vi "UHR-Fleezers Control (host) - 12.7c.vi"() -> ()   [LabVIEW 2012] (continued)
          }
          frame True {
            w4365 = TRUE ("AI to FIFO")
            n2420 = local read "Scan steps (MCL)"() -> (w4344:u64)
            n2421 = local read "Scan lines (y)"() -> (w4340:u64)
            n2422 = local read "Fast Scan Dir"() -> (w4351:bool)
            n2423 = local read "Actual MCL Inc (V)"() -> (w4341:dbl)
            n2424 = Decrement(x=w4340) -> (x-1=w4339:u64)
            n2425 = Decrement(x=w4344) -> (x-1=w4343:u64)
            n2426 = Multiply(x=w4341, y=w4339) -> (x*y=w4338:dbl)
            n2427 = Divide(x=w4338, y=2.0) -> (x/y=w4348:dbl)
            n2428 = Multiply(x=w4341, y=w4343) -> (x*y=w4342:dbl)
            n2429 = Divide(x=w4342, y=2.0) -> (x/y=w4347:dbl)
            n2430 = Select(t=w4347, s=w4351, f=w4348) -> (s? t:f=w4346:dbl)
            n2431 = Select(t=w4348, s=w4351, f=w4347) -> (s? t:f=w4350:dbl)
            n2432 = Subtract(x=w4358, y=w4350) -> (x-y=w4349:dbl)
            n2433 = Subtract(x=w4361, y=w4346) -> (x-y=w4345:dbl)
            n2434 = local read "2D or 1D Scan"() -> (w4363:bool)
            n2435 = Not(x=w4351) -> (.not. x?=w4357:bool)
            n2436 = Not(x=w4363) -> (.not. x?=w4359:bool)
            n2437 = And(x=w4351, y=w4359) -> (x .and. y?=w4360:bool)
            n2438 = And(x=w4359, y=w4357) -> (x .and. y?=w4362:bool)
            n2439 = Select(t=w4361, s=w4362, f=w4345) -> (s? t:f=w4352:dbl)
            n2440 = Select(t=w4358, s=w4360, f=w4349) -> (s? t:f=w4353:dbl)
            n2441 = call "Volt to I16.vi"("Voltage In"=w4353) -> ("I16 Voltage Out"=w4356:i16)
            n2442 = call "Volt to I16.vi"("Voltage In"=w4352) -> ("I16 Voltage Out"=w4355:i16)
            n2443 = xnode "Read/Write Control"("FPGA VI Reference In"=w4369, "error in"=w4368, "AI to FIFO"=w4365, "APD to FIFO"=w4365, "Start scan (MCL)"=w4365, "AO1"=w4356, "AO2"=w4355) -> ("FPGA VI Reference Out"=w4367:T20, "error out"=w4366:errorcluster)
          }
        }
        "Initial Y" <- w4318
        "Initial X" <- w4317
        n2444 = local write "Tab Control 6"(T3."Imaging" ("Tab Control 6")) -> ()
        "wait to reset values" <- w4319
      }
    }
    n2445 = local read "APD Elements/DMA read"() -> (w3471:u32)
    n2446 = local read "Trap AI Elements/DMA read"() -> (w3692:u32)
    n2447 = xnode "Get APD Data"("FPGA VI Reference In"=w3630, "error in"=w3629, "Number of Elements"=w3471, "Timeout (ms)"=-1) -> ("Data"=w3661:u32[], "Elements Remaining"=→"APD FIFO Elements Remaining":u32)  [unwired: 2 out]
    n2448 = local read "Trap Pos Elements/DMA read"() -> (w3626:u32)
    n2449 = xnode "Invoke Method"("FPGA VI Reference In"=w3630, "error in"=w3629, "Number of Elements"=w3626, "Timeout (ms)"=-1) -> ("Data"=w3590:u16[], "Elements Remaining"=→"Trap Pos FIFO El Remaining":u32)  [unwired: 2 out]
    n2450 = xnode "Get Trap Data"("FPGA VI Reference In"=w3630, "error in"=w3629, "Number of Elements"=w3692, "Timeout (ms)"=-1 ("Timeout")) -> ("FPGA VI Reference Out"=w3525:T20, "error out"=w3524:errorcluster, "Data"=w3591:i16[], "Elements Remaining"=w3815:u32)
    "FIFO El. Rem." <- w3815
    n2451 = local read "DMA Update Period (s)"() -> (w3693:dbl)
    n2452 = local read "Trap AI FIFO Depth"() -> (w3817:u32)
    n2453 = local read "Number of APDs"() -> (w3493:u8)
    n2454 = Decimate 1D Array(w3590) -> (w3587:u16[], w3589:u16[], w3588:u16[])
    n2455 = feedback #6(0.0) -> (w3619:dbl)
    n2456 = Add(x=w3693, y=w3619) -> (x+y=w3791:dbl)
    n2457 = feedback-in #6(w3791) -> ()
    n2458 = To Time Stamp(1:w3619) -> (0:w3618:timestamp)
    n2459 = Subtract(x=w3817, y=w3692) -> (x-y=w3816:u32)
    n2460 = To Unsigned Long Integer(number=w3587) -> (unsigned 32bit integer=w3586:u32[])
    n2461 = Join Numbers(hi=w3589, lo=w3588) -> ((hi.lo)=w3585:u32[])
    n2462 = Divide(x=w3815, y=w3816) -> (x/y=w3814:dbl)
    "Buffer Status" <- w3814
    n2463 = case "Deinterlace APD signals" shown="3, Default" w3493 {
      tunnel: [w3827 w3833] -> w3470
      tunnel: w3661 -> [w3828 w3832]
      tunnel: [w3826 w3831] -> w3469
      tunnel: [w3825 w3829] -> w3476
      frame 3, Default {
        n2464 = Decimate 1D Array "APD signals"(w3828) -> (w3827:u32[], w3826:u32[], w3825:u32[])
      }
      frame 2 {
        n2465 = Decimate 1D Array "APD signals"(w3832) -> (w3833:u32[], w3831:u32[])
        n2466 = Multiply(x=w3831, y=u32 0) -> (x*y=w3829:u32[])
      }
    }
    n2467 = Join Numbers(hi=w3586, lo=w3585) -> ((hi.lo)=w3579:u64[])
    n2468 = call "IR AOM word to freq - vec.vi"("Frequency Word In (double vec)"=w3579) -> ("Frequency Out"=w3625:dbl[])
    n2469 = Equal?(x=w3814, y=1.0) -> (x = y?=w3812:bool)
    n2470 = case "Alert buffer overflow" shown="True" w3812 {
      frame False {
      }
      frame True {
        n2471 = call <vilib>:"Beep.vi"() -> ()  [unwired: 3 in, 9 out]
        "Overflow (data lost)" <- TRUE ("Overflow (data lost)")
      }
    }
    n2472 = Decimate 1D Array(w3625) -> (w3624:dbl[], w3623:dbl[])
    n2473 = Build Array(w3624, w3623) -> (w3622:dbl[][])
    n2474 = Bundle(w3470, w3469, w3476) -> (w3474:cluster{u32[], u32[], u32[]})  [unwired: 1 in]
    n2475 = Build Array(w3470, w3469, w3476) -> (w3751:u32[][])
    n2476 = for {
      tunnel: w3470 -> [w3823] mode=indexing
      n2477 = call "Smart Buffer (DBL) 1.vi"("new element [write]"=w3823, "mode"=T21."write") -> ()  [unwired: 4 in, 6 out]
    }
    n2478 = local read "APD Integration Time (s)"() -> (w3486:dbl)
    n2479 = To Double Precision Float(number=w3751) -> (double precision float=w3752:dbl[][])
    n2480 = feedback #7 "APD3"(w3476) -> (w3492:u32[])
    n2481 = feedback #8 "APD2"(w3469) -> (w3648:u32[])
    n2482 = feedback #9 "APD1"(w3470) -> (w3750:u32[])
    n2483 = Build Array (concatenate)(w3648, w3469) -> (w3647:u32[])
    n2484 = Build Array (concatenate)(w3492, w3476) -> (w3491:u32[])
    n2485 = Build Array (concatenate)(w3750, w3470) -> (w3747:u32[])
    n2486 = for {
      tunnel: w3469 -> [w3822] mode=indexing
      n2487 = call "Smart Buffer (DBL) 2.vi"("new element [write]"=w3822, "mode"=T21."write") -> ()  [unwired: 4 in, 6 out]
    }
    n2488 = Array Size(array=w3747) -> (size(s)=w3744:i32)
    n2489 = Array Size(array=w3470) -> (size(s)=w3746:i32)
    n2490 = Multiply(x=w3746, y="APD Ave N") -> (x*y=w3745:dbl)
    n2491 = Greater?(x=w3744, y=w3745) -> (0:w3748:bool)
    n2492 = Bundle("APD 1", "APD 2", "APD 3") -> (w3784:cluster{string, string, string})  [unwired: 1 out]
    n2493 = local read "Trap Sets"() -> (w3691:u32)
    n2494 = case shown="True" w3748 {
      tunnel: w3747 -> [w4125 w4134]
      tunnel: [w4125 w4132] -> w3698
      tunnel: w3745 -> [_ w4127]
      tunnel: w3744 -> [_ w4133]
      tunnel: w3647 -> [w4124 w4131]
      tunnel: [w4124 w4130] -> w3645
      tunnel: w3491 -> [w4123 w4129]
      tunnel: [w4123 w4126] -> w3487
      frame False {
      }
      frame True {
        n2495 = Subtract(x=w4133, y=w4127) -> (x-y=w4128:dbl)
        n2496 = Array Subset "APD3"(array=w4129, index=w4128, length=w4127) -> (w4126:u32[])
        n2497 = Array Subset "APD2"(array=w4131, index=w4128, length=w4127) -> (w4130:u32[])
        n2498 = Array Subset "APD1"(array=w4134, index=w4128, length=w4127) -> (w4132:u32[])
      }
    }
    n2499 = feedback-in #7(w3487) -> ()
    n2500 = feedback-in #8(w3645) -> ()
    n2501 = feedback-in #9(w3698) -> ()
    n2502 = Cluster To Array(cluster=w3784) -> (array=w3781:string[])
    n2503 = for "APD" {
      tunnel: w3752 -> [w4381] mode=indexing
      tunnel: w3486 -> [w4388]
      tunnel: [w4384] -> w3649 mode=indexing
      tunnel: "APD Disp. Scale" -> [w4385]
      tunnel: w3781 -> [w4383] mode=indexing
      tunnel: "APD Disp. Downsample" -> [w4379]
      tunnel: [w4382] -> w3780
      workers-P: _ -> [_]
      tunnel: w3618 -> [w4378]
      n2504 = call "integrate 1D array interval - double.vi"("Ave N"=w4379, "Array In"=w4381) -> ("Array Out"=w4380:dbl[])  [unwired: 1 out]
      n2505 = Multiply(x=w4388, y=w4379) -> (x*y=w4382:dbl)
      n2506 = Divide(x=w4380, y=w4385) -> (x/y=w4386:dbl[])
      n2507 = Bundle By Name("t0"=w4378, "Y"=w4386, "dt"=w4382) -> (w4387:waveform(dbl))  [unwired: 1 out]
      n2508 = Set Waveform Attribute(5:w4383, 6:"NI_ChannelName" ("name"), 7:w4387) -> (3:w4384:waveform(dbl))  [unwired: 1 in, 2 out]
    }
    "APD Display Period (s)" <- w3780
    n2509 = Reciprocal(x=w3780) -> (1/x=→"APD Display Freq. (Hz)":dbl)
    n2510 = case "Deinterlace trap data, average down PSD" shown="2" w3691 {
      tunnel: w3591 -> [w4406 w4471]
      tunnel: [w4403 w4468] -> w3684
      tunnel: [w4406 w4470] -> w3582
      tunnel: "Detector Type" -> [w4405 w4466]
      tunnel: [w4404 w4469] -> w3683
      tunnel: [w4402 w4467] -> w3789
      frame 1, Default {
        n2511 = Divide(x=w4406, y=3276.7) -> (x/y=w4407:dbl[])
        n2512 = Decimate 1D Array(w4407) -> (w4416:dbl[], w4415:dbl[], w4414:dbl[], w4413:dbl[], w4412:dbl[], w4411:dbl[], w4410:dbl[], w4409:dbl[])
        n2513 = case shown="\"IR-QPD + PSD + FB-QPD position\"" w4405 {
          tunnel: w4416 -> [w4440 w4465]
          tunnel: w4415 -> [w4439 w4464]
          tunnel: w4414 -> [w4424 w4442]
          tunnel: w4413 -> [w4425 w4452]
          tunnel: w4412 -> [w4438 w4463]
          tunnel: w4411 -> [w4437 w4462]
          tunnel: w4410 -> [w4421 w4443]
          tunnel: w4409 -> [w4420 w4441]
          tunnel: [w4419 w4449] -> w4404
          tunnel: [w4418 w4448] -> w4403
          tunnel: [w4417 w4447] -> w4402
          frame "IR-QPD + PSD + FB-QPD", Default {
            w4417 = 0  # Channel pattern
            n2514 = Divide(x=w4440, y=w4425) -> (x/y=w4427:dbl[])
            n2515 = Divide(x=w4439, y=w4425) -> (x/y=w4426:dbl[])
            n2516 = Divide(x=w4438, y=w4421) -> (x/y=w4423:dbl[])
            n2517 = Divide(x=w4437, y=w4420) -> (x/y=w4422:dbl[])
            n2518 = Build Array(w4427, w4426, w4425, w4424, w4423, w4422, w4421, w4420) -> (w4418:dbl[][])
            n2519 = Bundle("T1 Y", "T1 X", "T1 Sum", "FB Sum", "PSD Y", "PSD X", "PSD Y Sum", "PSD X Sum") -> (w4436:T44)  [unwired: 1 out]
            n2520 = Cluster To Array(cluster=w4436) -> (array=w4419:string[])
          }
          frame "IR-QPD + PSD + FB-QPD position" {
            w4447 = 3  # Channel pattern
            n2521 = Negate(x=w4443) -> (-x=w4444:dbl[])
            n2522 = Divide(x=w4465, y=w4452) -> (x/y=w4454:dbl[])
            n2523 = Divide(x=w4464, y=w4452) -> (x/y=w4453:dbl[])
            n2524 = Divide(x=w4463, y=w4443) -> (x/y=w4451:dbl[])
            n2525 = Divide(x=w4462, y=w4444) -> (x/y=w4450:dbl[])
            n2526 = Build Array(w4454, w4453, w4452, w4441, w4442, w4451, w4450, w4443) -> (w4448:dbl[][])
            n2527 = Bundle("T1 Y", "T1 X", "T1 Sum", "FB X", "FB Sum", "PSD Y", "PSD X", "PSD Y Sum") -> (w4461:T44)  [unwired: 1 out]
            n2528 = Cluster To Array(cluster=w4461) -> (array=w4449:string[])
          }
        }
      }
      frame 2 {
        n2529 = case shown="\"IR-QPD + PSD + FB-QPD X position\"" w4466 {
          tunnel: w4471 -> [w4533 w4605 w4676]
          tunnel: [w4472 w4596 w4607] -> w4470
          tunnel: [w4499 w4587 w4654] -> w4469
          tunnel: [w4498 w4550 w4621] -> w4468
          tunnel: [w4492 w4585 w4652] -> w4467
          frame "IR-QPD + PSD + FB-QPD", Default {
            w4492 = 1  # Channel pattern
            # "time average x2 the 4th signal and the 4 psd signals (detection laser)"
            # "deinterlace 3 signals from qpd"
            n2530 = Decimate 1D Array(w4533) -> (w4532:i16[], w4531:i16[], w4497:i16[], w4530:i16[], w4520:i16[], w4518:i16[], w4517:i16[], w4515:i16[])
            n2531 = Decimate 1D Array(w4497) -> (w4496:i16[], w4495:i16[])
            n2532 = Decimate 1D Array(w4532) -> (w4529:i16[], w4501:i16[])
            n2533 = Decimate 1D Array(w4531) -> (w4528:i16[], w4526:i16[])
            n2534 = Decimate 1D Array(w4530) -> (w4527:i16[], w4525:i16[])
            n2535 = call "downsample 1D array - double.vi"("Ave N"=2.0, "Array In"=w4520) -> ("Array Out"=w4519:dbl[])  [unwired: 1 out]
            n2536 = call "downsample 1D array - double.vi"("Ave N"=2.0, "Array In"=w4518) -> ("Array Out"=w4500:dbl[])  [unwired: 1 out]
            n2537 = call "downsample 1D array - double.vi"("Ave N"=2.0, "Array In"=w4517) -> ("Array Out"=w4516:dbl[])  [unwired: 1 out]
            n2538 = call "downsample 1D array - double.vi"("Ave N"=2.0, "Array In"=w4515) -> ("Array Out"=w4514:dbl[])  [unwired: 1 out]
            n2539 = Interleave 1D Arrays(w4529, w4528, w4527, w4501, w4526, w4525, w4496, w4495, w4519, w4500, w4516, w4514) -> (w4513:dbl[])
            n2540 = Divide(x=w4513, y=3276.7) -> (x/y=w4512:dbl[])
            n2541 = Decimate 1D Array(w4512) -> (w4511:dbl[], w4510:dbl[], w4509:dbl[], w4508:dbl[], w4507:dbl[], w4506:dbl[], w4494:dbl[], w4493:dbl[], w4505:dbl[], w4504:dbl[], w4503:dbl[], w4502:dbl[])
            n2542 = Divide(x=w4511, y=w4509) -> (x/y=w4479:dbl[])
            n2543 = Divide(x=w4510, y=w4509) -> (x/y=w4478:dbl[])
            n2544 = Divide(x=w4508, y=w4506) -> (x/y=w4477:dbl[])
            n2545 = Divide(x=w4507, y=w4506) -> (x/y=w4476:dbl[])
            n2546 = Divide(x=w4505, y=w4503) -> (x/y=w4475:dbl[])
            n2547 = Divide(x=w4504, y=w4502) -> (x/y=w4474:dbl[])
            n2548 = Build Array(w4479, w4478, w4509, w4477, w4476, w4506, w4494, w4493, w4475, w4474, w4503, w4502) -> (w4498:dbl[][])
            n2549 = Bundle("T1 Y", "T1 X", "T1 Sum", "T2 Y", "T2 X", "T2 Sum", "T1 FB Sum", "T2 FB Sum", "PSD Y", "PSD X", "PSD Y Sum", "PSD X Sum") -> (w4480:T45)  [unwired: 1 out]
            n2550 = To Word Integer(number=w4513) -> (16bit integer=w4472:i16[])
            n2551 = Cluster To Array(cluster=w4480) -> (array=w4499:string[])
          }
          frame "IR-QPD + PSD + FB-QPD X position" {
            w4585 = 2  # Channel pattern
            # "time average x2 the 3 psd signals (detection laser)"
            # "deinterlace 3 signals from qpds"
            n2552 = Decimate 1D Array(w4605) -> (w4604:i16[], w4603:i16[], w4586:i16[], w4602:i16[], w4548:i16[], w4545:i16[], w4542:i16[], w4573:i16[])
            n2553 = Select(t=i16 -1, s="Flip X Sign", f=i16 1) -> (s? t:f=w4538:i16)
            n2554 = Multiply(x=w4603, y=w4538) -> (x*y=w4539:i16[])
            n2555 = Decimate 1D Array(w4586) -> (w4571:i16[], w4569:i16[])
            n2556 = Decimate 1D Array(w4604) -> (w4601:i16[], w4588:i16[])
            n2557 = Decimate 1D Array(w4539) -> (w4600:i16[], w4598:i16[])
            n2558 = Decimate 1D Array(w4602) -> (w4599:i16[], w4597:i16[])
            n2559 = Decimate 1D Array(w4573) -> (w4572:i16[], w4570:i16[])
            n2560 = call "downsample 1D array - I16.vi"("Ave N"=2.0, "Array In"=w4548) -> ("Array Out"=w4546:i16[])  [unwired: 1 in]
            n2561 = call "downsample 1D array - I16.vi"("Ave N"=2.0, "Array In"=w4542) -> ("Array Out"=w4540:i16[])  [unwired: 1 in]
            n2562 = call "downsample 1D array - I16.vi"("Ave N"=2.0, "Array In"=w4545) -> ("Array Out"=w4543:i16[])  [unwired: 1 in]
            n2563 = Interleave 1D Arrays(w4601, w4600, w4599, w4588, w4598, w4597, w4572, w4571, w4570, w4569, w4546, w4543, w4540) -> (w4596:i16[])
            n2564 = Divide(x=w4596, y=3276.7) -> (x/y=w4595:dbl[])
            n2565 = Decimate 1D Array(w4595) -> (w4594:dbl[], w4593:dbl[], w4592:dbl[], w4591:dbl[], w4590:dbl[], w4589:dbl[], w4561:dbl[], w4559:dbl[], w4558:dbl[], w4556:dbl[], w4555:dbl[], w4554:dbl[], w4551:dbl[])
            n2566 = Negate(x=w4551) -> (-x=w4549:dbl[])
            n2567 = Divide(x=w4555, y=w4551) -> (x/y=w4553:dbl[])
            n2568 = Divide(x=w4554, y=w4549) -> (x/y=w4552:dbl[])
            n2569 = Divide(x=w4594, y=w4592) -> (x/y=w4577:dbl[])
            n2570 = Divide(x=w4593, y=w4592) -> (x/y=w4576:dbl[])
            n2571 = Divide(x=w4591, y=w4589) -> (x/y=w4575:dbl[])
            n2572 = Divide(x=w4590, y=w4589) -> (x/y=w4574:dbl[])
            n2573 = Divide(x=w4561, y=w4559) -> (x/y=w4560:dbl[])
            n2574 = Divide(x=w4558, y=w4556) -> (x/y=w4557:dbl[])
            n2575 = Build Array(w4577, w4576, w4592, w4575, w4574, w4589, w4560, w4559, w4557, w4556, w4553, w4552, w4551) -> (w4550:dbl[][])
            n2576 = Bundle("T1 Y", "T1 X", "T1 Sum", "T2 Y", "T2 X", "T2 Sum", "T1 FB X", "T1 FB Sum", "T2 FB X", "T2 FB Sum", "PSD Y", "PSD X", "PSD Y Sum") -> (w4578:T46)  [unwired: 1 out]
            n2577 = Cluster To Array(cluster=w4578) -> (array=w4587:string[])
          }
          frame "IR-QPD + PSD + FB-QPD XY positions" {
            w4652 = 4  # Channel pattern
            # "time average x2 the 3 psd signals (detection laser)"
            # "deinterlace 3 signals from qpds"
            n2578 = Decimate 1D Array(w4676) -> (w4675:i16[], w4674:i16[], w4653:i16[], w4673:i16[], w4619:i16[], w4665:i16[], w4664:i16[], w4641:i16[])
            n2579 = Decimate 1D Array "Feedback Sum"(w4653) -> (w4637:i16[], w4635:i16[])
            n2580 = Decimate 1D Array "QPD Y"(w4675) -> (w4672:i16[], w4655:i16[])
            n2581 = Decimate 1D Array "QPD X"(w4674) -> (w4671:i16[], w4669:i16[])
            n2582 = Decimate 1D Array "Feedback Y"(w4619) -> (w4618:i16[], w4617:i16[])
            n2583 = Decimate 1D Array "QPD Sum"(w4673) -> (w4670:i16[], w4668:i16[])
            n2584 = Decimate 1D Array "Feedback X"(w4641) -> (w4638:i16[], w4636:i16[])
            n2585 = call "downsample 1D array - double.vi"("Ave N"=2.0, "Array In"=w4665) -> ("Array Out"=w4640:dbl[])  [unwired: 1 out]
            n2586 = call "downsample 1D array - double.vi"("Ave N"=2.0, "Array In"=w4664) -> ("Array Out"=w4639:dbl[])  [unwired: 1 out]
            n2587 = Interleave 1D Arrays(w4672, w4671, w4670, w4655, w4669, w4668, w4618, w4638, w4637, w4617, w4636, w4635, w4640, w4639) -> (w4663:dbl[])
            n2588 = Divide(x=w4663, y=3276.7) -> (x/y=w4662:dbl[])
            n2589 = Decimate 1D Array(w4662) -> (w4661:dbl[], w4660:dbl[], w4659:dbl[], w4658:dbl[], w4657:dbl[], w4656:dbl[], w4614:dbl[], w4628:dbl[], w4612:dbl[], w4613:dbl[], w4626:dbl[], w4610:dbl[], w4624:dbl[], w4622:dbl[])
            n2590 = Negate(x=w4622) -> (-x=w4620:dbl[])
            n2591 = Divide(x=w4624, y=w4620) -> (x/y=w4623:dbl[])
            n2592 = Divide(x=w4613, y=w4610) -> (x/y=w4609:dbl[])
            n2593 = Divide(x=w4614, y=w4612) -> (x/y=w4611:dbl[])
            n2594 = Divide(x=w4661, y=w4659) -> (x/y=w4645:dbl[])
            n2595 = Divide(x=w4660, y=w4659) -> (x/y=w4644:dbl[])
            n2596 = Divide(x=w4658, y=w4656) -> (x/y=w4643:dbl[])
            n2597 = Divide(x=w4657, y=w4656) -> (x/y=w4642:dbl[])
            n2598 = Divide(x=w4628, y=w4612) -> (x/y=w4627:dbl[])
            n2599 = Divide(x=w4626, y=w4610) -> (x/y=w4625:dbl[])
            n2600 = Build Array(w4645, w4644, w4659, w4643, w4642, w4656, w4611, w4627, w4612, w4609, w4625, w4610, w4623, w4622) -> (w4621:dbl[][])
            n2601 = Bundle("T1 Y", "T1 X", "T1 Sum", "T2 Y", "T2 X", "T2 Sum", "T1 FB Y", "T1 FB X", "T1 FB Sum", "T2 FB Y", "T2 FB X", "T2 FB Sum", "PSD X", "PSD Y Sum") -> (w4608:T47)  [unwired: 1 out]
            n2602 = To Word Integer(number=w4663) -> (16bit integer=w4607:i16[])
            n2603 = Cluster To Array(cluster=w4608) -> (array=w4654:string[])
          }
        }
      }
    }
    "AI labels" <- w3683
    n2604 = local read "APD Integration Time (s)"() -> (w3656:dbl)
    n2605 = Array Size(array=w3698) -> (size(s)=w3743:i32)
    n2606 = call <vilib>:"Std Deviation and Variance.vi"("X"=w3645) -> ("standard deviation"=w3644:dbl)  [unwired: 1 in, 2 out]
    n2607 = Add Array Elements(numeric array=w3645) -> (sum=w3646:u32)
    n2608 = Add Array Elements(numeric array=w3698) -> (sum=w3753:u32)
    n2609 = call <vilib>:"Std Deviation and Variance.vi"("X"=w3698) -> ("standard deviation"=w3697:dbl)  [unwired: 1 in, 2 out]
    n2610 = Divide(x=w3644, y=w3486) -> (x/y=w3641:dbl)
    "Rate sigma (Hz) 2" <- w3641
    n2611 = Multiply(x=w3486, y=w3743) -> (x*y=w3488:dbl)
    "Int. Time (s)" <- w3488
    n2612 = Divide(x=w3646, y=w3488) -> (x/y=w3642:dbl)
    "APD 2 Rate (Hz)" <- w3642
    n2613 = Multiply(x="APD Disp. Scale", y=w3649) -> (x*y=w3658:waveform(dbl)[])
    n2614 = Divide(x=w3753, y=w3488) -> (x/y=w3695:dbl)
    "APD 1 Rate (Hz)" <- w3695
    n2615 = Divide(x=w3697, y=w3486) -> (x/y=w3696:dbl)
    "Rate sigma (Hz)" <- w3696
    n2616 = Divide(x=w3641, y=w3642) -> (x/y=→"Sigma/Mean 2":dbl)
    n2617 = Multiply(x="APD Disp. Downsample", y=w3656) -> (x*y=w3654:dbl)
    n2618 = Divide(x=w3696, y=w3695) -> (x/y=→"Sigma/Mean":dbl)
    n2619 = Divide(x=w3658, y=w3654) -> (x/y=w3478:waveform(dbl)[])
    n2620 = Index Array(array=w3478, index=0) -> (element=w3638:waveform(dbl))
    n2621 = Index Array(array=w3478, index=1) -> (element=w3636:waveform(dbl))
    n2622 = Index Array(array=w3478, index=2) -> (element=w3480:waveform(dbl))
    n2623 = Subtract(x=w3638, y="APD 1 Offset") -> (x-y=w3634:waveform(dbl))
    n2624 = Subtract(x=w3636, y="APD 2 Offset") -> (x-y=w3633:waveform(dbl))
    n2625 = Subtract(x=w3480, y="APD 3 Offset") -> (x-y=w3477:waveform(dbl))
    n2626 = Add Array Elements(numeric array=w3487) -> (sum=w3490:u32)
    n2627 = call <vilib>:"Std Deviation and Variance.vi"("X"=w3487) -> ("standard deviation"=w3489:dbl)  [unwired: 1 in, 2 out]
    n2628 = Build Array(w3634, w3633, w3477) -> (→"APD Chart":waveform(dbl)[])
    n2629 = Divide(x=w3490, y=w3488) -> (x/y=w3484:dbl)
    "APD 3 Rate (Hz)" <- w3484
    n2630 = Divide(x=w3489, y=w3486) -> (x/y=w3485:dbl)
    "Rate sigma (Hz) 3" <- w3485
    n2631 = Divide(x=w3485, y=w3484) -> (x/y=→"Sigma/Mean 3":dbl)
    n2632 = local read "Data Period (s)"() -> (w3541:dbl)
    n2633 = local read "BD 1 Frequency 2 (MHz)"() -> (w3574:dbl)
    n2634 = local read "BD 1 Frequency 1 (MHz)"() -> (w3575:dbl)
    n2635 = Decimate 1D Array(w3582) -> (w3606:i16[], w3605:i16[], w3603:i16[], w3602:i16[])  [unwired: 9 out]
    n2636 = Multiply(x=w3541, y="Trap Pos. Disp. Downsample") -> (x*y=w3539:dbl)
    n2637 = Divide(x=w3606, y=w3605) -> (x/y=w3607:dbl[])
    n2638 = Divide(x=w3603, y=w3602) -> (x/y=w3604:dbl[])
    n2639 = local read "AOM X Cal (nm/MHz)"() -> (w3572:dbl)
    n2640 = Split 1D Array(array=w3607, index="N El. to Ave.") -> (second subarray=w3610:dbl[])  [unwired: 1 out]
    n2641 = Split 1D Array(array=w3604, index="N El. to Ave.") -> (second subarray=w3609:dbl[])  [unwired: 1 out]
    n2642 = Multiply(x=w3541, y="Trap Disp. Downsample") -> (x*y=w3620:dbl)
    "Display Period (s)" <- w3620
    n2643 = for "Trap AI" {
      tunnel: [w4401] -> w3785 mode=indexing
      tunnel: w3618 -> [w4392]
      tunnel: "Trap Disp. Downsample" -> [w4399]
      tunnel: w3684 -> [w4397] mode=indexing
      tunnel: w3541 -> [w4396]
      tunnel: w3683 -> [w4395] mode=indexing
      tunnel: [w4394] -> w3653 mode=indexing
      tunnel: w3620 -> [w4393]
      workers-P: _ -> [_]
      n2644 = Bundle By Name("Y"=w4397, "dt"=w4396) -> (w4398:waveform(dbl))  [unwired: 1 out]
      n2645 = Set Waveform Attribute(5:w4395, 6:"NI_ChannelName" ("name"), 7:w4398) -> (3:w4394:waveform(dbl))  [unwired: 1 in, 2 out]
      n2646 = call "downsample 1D array - double.vi"("Ave N"=w4399, "Array In"=w4397) -> ("Array Out"=w4400:dbl[])  [unwired: 1 out]
      n2647 = Bundle By Name(cluster=w4394, "t0"=w4392, "Y"=w4400, "dt"=w4393) -> (w4401:waveform(dbl))
    }
    n2648 = Bundle("BD 1 Frequency 1 (MHz)"=w3575, "BD 1 Frequency 2 (MHz)"=w3574) -> (w3576:T48)  [unwired: 1 out]
    n2649 = call-poly <vilib>:"Mean.vi"("X"=w3609) -> ("mean"=w3597:dbl)  [unwired: 1 out]
    n2650 = call-poly <vilib>:"Mean.vi"("X"=w3610) -> ("mean"=w3598:dbl)  [unwired: 1 out]
    n2651 = Reciprocal(x=w3620) -> (1/x=→"Trap Disp. Freq. (Hz)":dbl)
    n2652 = Cluster To Array(cluster=w3576) -> (array=w3573:dbl[])
    n2653 = local read "Trap X AI1 (DMA)"() -> (w3608:T13)
    n2654 = local read "Data points/scans (MCL)"() -> (w3763:dbl)
    n2655 = To Fixed-Point(number=w3597) -> (fixed-point=w3595:fxp<+/-,16,1>)  [unwired: 1 in]
    n2656 = To Fixed-Point(number=w3598) -> (fixed-point=w3596:fxp<+/-,16,1>)  [unwired: 1 in]
    n2657 = Bundle("Trap 1 Pos.", "Trap 2 Pos.") -> (w3617:cluster{string, string})  [unwired: 1 out]
    n2658 = Bundle By Name(cluster=w3608, "Set 1"=w3596, "Set 2"=w3595) -> (→"Trap X AI1 (DMA)":T13)
    n2659 = Cluster To Array(cluster=w3617) -> (array=w3614:string[])
    n2660 = Unbundle(w3474) -> (w3475:u32[])  [unwired: 2 out]
    n2661 = Select(t=-1.0, s="Negate Y Axis", f=1.0) -> (s? t:f=w3558:dbl)
    n2662 = for "Trap Position" {
      tunnel: w3622 -> [w3993] mode=indexing
      tunnel: "Trap Pos. Disp. Downsample" -> [w3992]
      tunnel: w3539 -> [w3990]
      tunnel: w3618 -> [w3989]
      tunnel: w3614 -> [w3987] mode=indexing
      tunnel: [w3986] -> w3528 mode=indexing
      tunnel: w3573 -> [w3984] mode=indexing
      tunnel: w3572 -> [w3982]
      tunnel: w3558 -> [w3981]
      n2663 = call "downsample 1D array - double.vi"("Ave N"=w3992, "Array In"=w3993) -> ("Array Out"=w3991:dbl[])  [unwired: 1 out]
      n2664 = Subtract(x=w3991, y=w3984) -> (x-y=w3985:dbl[])
      n2665 = Multiply(x=w3982, y=w3985) -> (x*y=w3983:dbl[])
      n2666 = Multiply(x=w3981, y=w3983) -> (x*y=w3980:dbl[])
      n2667 = Bundle By Name("Y"=w3980, "dt"=w3990, "t0"=w3989) -> (w3988:waveform(dbl))  [unwired: 1 out]
      n2668 = Set Waveform Attribute(5:w3987, 6:"NI_ChannelName" ("name"), 7:w3988) -> (3:w3986:waveform(dbl))  [unwired: 1 in, 2 out]
    }
    n2669 = To Double Precision Float(number=w3475) -> (double precision float=w3681:dbl[])
    n2670 = local read "Display Period (s)"() -> (w3670:dbl)
    n2671 = Increment(x=w3763) -> (x+1=w3764:dbl)
    n2672 = Index Array(array=w3528, index=0) -> (element=w3532:waveform(dbl))
    n2673 = Index Array(array=w3528, index=1) -> (element=w3527:waveform(dbl))
    n2674 = feedback #10(w3764) -> (w3767:dbl)
    n2675 = Select(t=0, s=w3754, f=w3767) -> (s? t:f=w3760:dbl)
    n2676 = Array Size(array=w3681) -> (size(s)=w3766:i32)
    n2677 = Build Array (concatenate)(w3649, w3785) -> (w3651:waveform(dbl)[])
    "All Signals" <- w3651
    n2678 = Add(x=w3766, y=w3760) -> (x+y=w3761:dbl)
    n2679 = Unbundle By Name(w3532) -> ("Y"=w3533:dbl[])
    n2680 = Divide(x="Bead Sep. Int. Time (s)", y=w3670) -> (x/y=w3568:dbl)
    n2681 = Add(x=w3533, y="FB Trap Pos Offset") -> (x+y=w3531:dbl[])
    "T1 x pos data" <- w3531
    n2682 = Greater?(x=w3761, y=w3763) -> (0:w3762:bool)
    n2683 = feedback #11(w3531) -> (w3570:dbl[])
    n2684 = Build Array (concatenate)(w3531, w3570) -> (w3569:dbl[])
    n2685 = Bundle By Name(cluster=w3532, "Y"=w3531) -> (w3530:waveform(dbl))
    n2686 = Select(t=w3760, s=w3762, f=w3761) -> (s? t:f=w3759:dbl)
    n2687 = feedback-in #10(w3759) -> ()
    n2688 = local read "MCL Scanning"() -> (w3757:bool)
    n2689 = Bundle(w3530, w3527) -> (w3526:cluster{waveform(dbl), waveform(dbl)})  [unwired: 1 out]
    n2690 = Split 1D Array(array=w3569, index=w3568) -> (first subarray=w3562:dbl[])  [unwired: 1 out]
    n2691 = feedback-in #11(w3562) -> ()
    n2692 = Not(x=w3762) -> (.not. x?=w3756:bool)
    n2693 = Cluster To Array(cluster=w3526) -> (array=w3502:waveform(dbl)[])
    "Trap Positions" <- w3502
    n2694 = call-poly <vilib>:"Mean.vi"("X"=w3562) -> ("mean"=w3561:dbl)  [unwired: 1 out]
    "Mean T1 Position (nm)" <- w3561
    n2695 = Subtract(x=w3562, y=w3561) -> (x-y=w3567:dbl[])
    n2696 = Square(x=w3567) -> (x^2=w3566:dbl[])
    n2697 = And(x=w3756, y=w3757) -> (x .and. y?=w3758:bool)
    n2698 = call-poly <vilib>:"Mean.vi"("X"=w3566) -> ("mean"=w3565:dbl)  [unwired: 1 out]
    n2699 = Square Root(x=w3565) -> (sqrt(x)=w3564:dbl)
    n2700 = Or(x=w3758, y=w3754) -> (x .or. y?=w3755:bool)
    n2701 = Equal?(x="Tab Control 6", y=T38."High Res Display") -> (x = y?=w3687:bool)
    n2702 = Multiply(x=10.0, y=w3564) -> (x*y=→"Trap 1 Position RMS (A)":dbl)
    n2703 = case "For displaying the high resolution display (no downsampling)" shown="True" w3687 {
      tunnel: w3653 -> [_ w4013]
      frame False {
      }
      frame True {
        n2704 = Index Array(array=w4013, index="High Res. Display") -> (element=w4014:waveform(dbl))
        n2705 = call <vilib>:"Std Deviation and Variance.vi"("X"=w4014) -> ("mean"=w4021:dbl, "standard deviation"=w4026:dbl)  [unwired: 1 in, 1 out]
        "Mean Intensity" <- w4021
        "Sigma" <- w4026
        n2706 = Subtract(x=w4014, y=w4021) -> (x-y=w4020:waveform(dbl))
        n2707 = Select(t=w4020, s="Subtract mean", f=w4014) -> (s? t:f=→"1 Channel":waveform(dbl))
        n2708 = Divide(x=w4026, y=w4021) -> (x/y=→"Sigma/Mean":dbl)
        n2709 = feedback #12(1) -> (w4015:i32)
        n2710 = Greater Or Equal?(x=w4015, y="Slow mean N ave.") -> (x >= y?=w4028:bool)
        n2711 = Increment(x=w4015) -> (x+1=w4030:i32)
        n2712 = Select(t=1, s=w4028, f=w4030) -> (s? t:f=w4017:i32)
        n2713 = feedback-in #12(w4017) -> ()
        n2714 = feedback #13() -> (w4018:waveform(dbl))  [unwired: 1 out]
        n2715 = case shown="Default" w4015 {
          tunnel: [w4033 w4036] -> w4019
          tunnel: w4018 -> [w4035 _]
          tunnel: w4014 -> [w4034 w4036]
          frame Default {
            n2716 = call-poly <vilib>:"Append Waveforms.vi"("waveform B"=w4034, "waveform A"=w4035) -> ("waveform out"=w4033:waveform(dbl))  [unwired: 1 in, 8 out]
          }
          frame 1 {
          }
        }
        n2717 = feedback-in #13(w4019) -> ()
        n2718 = case shown="True" w4028 {
          tunnel: w4019 -> [_ w4032]
          frame False {
          }
          frame True {
            n2719 = call-poly <vilib>:"Mean.vi"("X"=w4032) -> ("mean"=→"Slow mean":dbl)  [unwired: 1 out]
          }
        }
      }
    }
    n2720 = case "For plotting results of scanning MCL (fluorescence and detection laser images)" shown="True" w3755 {
      tunnel: w3754 -> [_ w4140]
      tunnel: w3763 -> [_ _]
      tunnel: w3653 -> [_ w4269]
      tunnel: w3631 -> [_ w4177]
      tunnel: w3474 -> [_ w4147]
      frame False {
      }
      frame True {
        w4157 = u32 0 items=["Horizontal", "Vertical", "Central", "1st Diagonal", "2nd Diagonal"] ("Type of Symmetry")
        w4184 = u32 0 items=["Horizontal", "Vertical", "Central", "1st Diagonal", "2nd Diagonal"] ("Type of Symmetry")
        w4208 = u32 0 items=["Horizontal", "Vertical", "Central", "1st Diagonal", "2nd Diagonal"] ("Type of Symmetry")
        w4211 = u32 0 items=["Horizontal", "Vertical", "Central", "1st Diagonal", "2nd Diagonal"] ("Type of Symmetry")
        w4240 = u32 0 items=["Horizontal", "Vertical", "Central", "1st Diagonal", "2nd Diagonal"] ("Type of Symmetry")
        n2721 = Unbundle(w4147) -> (w4146:u32[], w4144:u32[], w4142:u32[])
        n2722 = To Double Precision Float(number=w4146) -> (double precision float=w4145:dbl[])
        n2723 = To Double Precision Float(number=w4144) -> (double precision float=w4143:dbl[])
        n2724 = To Double Precision Float(number=w4142) -> (double precision float=w4141:dbl[])
        n2725 = Index Array(array=w4269, index=10) -> (element=w4275:waveform(dbl))
        n2726 = Index Array(array=w4269, index=11) -> (element=w4272:waveform(dbl))
        n2727 = local read "Cycles/step (MCL)"() -> (w4225:u64)
        n2728 = Index Array(array=w4269, index="Channel") -> (element=w4271:waveform(dbl))
        n2729 = Unbundle(w4177) -> ("New Image"=w4176:T2, "New Image"=w4175:T2, "New Image"=w4148:T2, "New Image"=w4149:T2, "New Image"=w4150:T2)
        n2730 = local read "Scan steps (MCL)"() -> (w4136:u64)
        n2731 = Unbundle By Name(w4275) -> ("Y"=w4227:dbl[])
        n2732 = Unbundle By Name(w4272) -> ("Y"=w4229:dbl[])
        n2733 = local read "Scan lines (y)"() -> (w4137:u64)
        n2734 = local read "N APD Samp/step"() -> (w4139:dbl)
        n2735 = Unbundle By Name(w4271) -> ("Y"=w4234:dbl[])
        n2736 = call "downsample 1D array - double.vi"("Ave N"=w4225, "Array In"=w4227) -> ("Array Out"=w4226:dbl[])  [unwired: 1 out]
        n2737 = call "downsample 1D array - double.vi"("Ave N"=w4225, "Array In"=w4229) -> ("Array Out"=w4228:dbl[])  [unwired: 1 out]
        n2738 = call "downsample 1D array - double.vi"("Ave N"=w4225, "Array In"=w4234) -> ("Array Out"=w4233:dbl[])  [unwired: 1 out]
        n2739 = Multiply(x=w4136, y=u64 2) -> (x*y=w4138:u64)
        n2740 = feedback #14(w4143) -> (w4202:dbl[])
        n2741 = Build Array (concatenate)(w4202, w4143) -> (w4201:dbl[])
        n2742 = feedback #15(w4141) -> (w4174:dbl[])
        n2743 = Build Array (concatenate)(w4174, w4141) -> (w4135:dbl[])
        n2744 = Select(t=w4143, s=w4140, f=w4201) -> (s? t:f=w4186:dbl[])
        n2745 = feedback-in #14(w4186) -> ()
        n2746 = Select(t=w4141, s=w4140, f=w4135) -> (s? t:f=w4159:dbl[])
        n2747 = feedback-in #15(w4159) -> ()
        n2748 = feedback #16(w4145) -> (w4295:dbl[])
        n2749 = Build Array (concatenate)(w4295, w4145) -> (w4277:dbl[])
        n2750 = Select(t=w4145, s=w4140, f=w4277) -> (s? t:f=w4281:dbl[])
        n2751 = feedback-in #16(w4281) -> ()
        n2752 = feedback #17(w4226) -> (w4283:dbl[])
        n2753 = Build Array (concatenate)(w4283, w4226) -> (w4274:dbl[])
        n2754 = feedback #18(w4233) -> (w4293:dbl[])
        n2755 = Build Array (concatenate)(w4293, w4233) -> (w4292:dbl[])
        n2756 = feedback #19(w4228) -> (w4285:dbl[])
        n2757 = Build Array (concatenate)(w4285, w4228) -> (w4286:dbl[])
        n2758 = Select(t=w4226, s=w4140, f=w4274) -> (s? t:f=w4230:dbl[])
        n2759 = feedback-in #17(w4230) -> ()
        n2760 = Select(t=w4233, s=w4140, f=w4292) -> (s? t:f=w4232:dbl[])
        n2761 = feedback-in #18(w4232) -> ()
        n2762 = Select(t=w4228, s=w4140, f=w4286) -> (s? t:f=w4231:dbl[])
        n2763 = feedback-in #19(w4231) -> ()
        n2764 = call "integrate 1D array interval - double.vi"("Ave N"=w4139, "Array In"=w4186) -> ("Array Out"=w4197:dbl[])  [unwired: 1 out]
        n2765 = call "integrate 1D array interval - double.vi"("Ave N"=w4139, "Array In"=w4159) -> ("Array Out"=w4170:dbl[])  [unwired: 1 out]
        n2766 = call "integrate 1D array interval - double.vi"("Ave N"=w4139, "Array In"=w4281) -> ("Array Out"=w4280:dbl[])  [unwired: 1 out]
        n2767 = Array Size(array=w4197) -> (size(s)=w4198:i32)
        n2768 = Array Size(array=w4170) -> (size(s)=w4171:i32)
        n2769 = Array Size(array=w4280) -> (size(s)=w4282:i32)
        n2770 = Multiply(x=w4137, y=w4138) -> (x*y=w4200:u64)
        n2771 = Multiply(x=w4137, y=w4138) -> (x*y=w4173:u64)
        n2772 = Multiply(x=w4137, y=w4138) -> (x*y=w4290:u64)
        n2773 = Subtract(x=w4200, y=w4198) -> (x-y=w4191:u64)
        n2774 = call-poly <vilib>:"Mean.vi"("X"=w4197) -> ("mean"=w4188:dbl)  [unwired: 1 out]
        n2775 = Subtract(x=w4173, y=w4171) -> (x-y=w4164:u64)
        n2776 = call-poly <vilib>:"Mean.vi"("X"=w4170) -> ("mean"=w4161:dbl)  [unwired: 1 out]
        n2777 = Subtract(x=w4290, y=w4282) -> (x-y=w4224:u64)
        n2778 = call-poly <vilib>:"Mean.vi"("X"=w4280) -> ("mean"=w4221:dbl)  [unwired: 1 out]
        n2779 = call-poly <vilib>:"Mean.vi"("X"=w4230) -> ("mean"=w4214:dbl)  [unwired: 1 out]
        n2780 = call-poly <vilib>:"Mean.vi"("X"=w4232) -> ("mean"=w4219:dbl)  [unwired: 1 out]
        n2781 = call-poly <vilib>:"Mean.vi"("X"=w4231) -> ("mean"=w4217:dbl)  [unwired: 1 out]
        n2782 = Initialize Array(1.0 ("element"), w4191) -> (w4187:dbl[])
        n2783 = Initialize Array(1.0 ("element"), w4164) -> (w4160:dbl[])
        n2784 = Initialize Array(1.0 ("element"), w4224) -> (w4215:dbl[])
        n2785 = Multiply(x=w4187, y=w4188) -> (x*y=w4189:dbl[])
        n2786 = Multiply(x=w4160, y=w4161) -> (x*y=w4162:dbl[])
        n2787 = Multiply(x=w4215, y=w4221) -> (x*y=w4222:dbl[])
        n2788 = Multiply(x=w4215, y=w4217) -> (x*y=w4218:dbl[])
        n2789 = Multiply(x=w4215, y=w4219) -> (x*y=w4220:dbl[])
        n2790 = Multiply(x=w4215, y=w4214) -> (x*y=w4216:dbl[])
        n2791 = Build Array (concatenate)(w4197, w4189) -> (w4199:dbl[])
        n2792 = Build Array (concatenate)(w4170, w4162) -> (w4172:dbl[])
        n2793 = Build Array (concatenate)(w4280, w4222) -> (w4289:dbl[])
        n2794 = Build Array (concatenate)(w4230, w4216) -> (w4284:dbl[])
        n2795 = Build Array (concatenate)(w4232, w4220) -> (w4288:dbl[])
        n2796 = Build Array (concatenate)(w4231, w4218) -> (w4287:dbl[])
        n2797 = Reshape Array(w4199, w4137, w4138) -> (w4195:dbl[][])
        n2798 = Reshape Array(w4172, w4137, w4138) -> (w4168:dbl[][])
        n2799 = Reshape Array(w4289, w4137, w4138) -> (w4267:dbl[][])
        n2800 = Reshape Array(w4284, w4137, w4138) -> (w4250:dbl[][])
        n2801 = Reshape Array(w4288, w4137, w4138) -> (w4242:dbl[][])
        n2802 = Reshape Array(w4287, w4137, w4138) -> (w4257:dbl[][])
        n2803 = Array Subset(array=w4195, index (col)=0 ("index"), length (col)=w4136) -> (w4194:dbl[][])  [unwired: 2 in]
        n2804 = Array Subset(array=w4195, index (col)=w4136) -> (w4192:dbl[][])  [unwired: 3 in]
        n2805 = Array Subset(array=w4168, index (col)=0 ("index"), length (col)=w4136) -> (w4167:dbl[][])  [unwired: 2 in]
        n2806 = Array Subset(array=w4168, index (col)=w4136) -> (w4165:dbl[][])  [unwired: 3 in]
        n2807 = Array Subset(array=w4257, index (col)=0 ("index"), length (col)=w4136) -> (w4262:dbl[][])  [unwired: 2 in]
        n2808 = Array Subset(array=w4257, index (col)=w4136) -> (w4260:dbl[][])  [unwired: 3 in]
        n2809 = Array Subset(array=w4267, index (col)=0 ("index"), length (col)=w4136) -> (w4266:dbl[][])  [unwired: 2 in]
        n2810 = Array Subset(array=w4267, index (col)=w4136) -> (w4264:dbl[][])  [unwired: 3 in]
        n2811 = Array Subset(array=w4242, index (col)=0 ("index"), length (col)=w4136) -> (w4248:dbl[][])  [unwired: 2 in]
        n2812 = Array Subset(array=w4242, index (col)=w4136) -> (w4246:dbl[][])  [unwired: 3 in]
        n2813 = Array Subset(array=w4250, index (col)=0 ("index"), length (col)=w4136) -> (w4255:dbl[][])  [unwired: 2 in]
        n2814 = Array Subset(array=w4250, index (col)=w4136) -> (w4253:dbl[][])  [unwired: 3 in]
        n2815 = for {
          tunnel: w4194 -> [w4299] mode=indexing
          tunnel: [w4298] -> w4193 mode=indexing
          workers-P: _ -> [_]
          n2816 = Reverse 1D Array(array=w4299) -> (reversed array=w4298:dbl[])
        }
        n2817 = for {
          tunnel: w4167 -> [w4297] mode=indexing
          tunnel: [w4296] -> w4166 mode=indexing
          workers-P: _ -> [_]
          n2818 = Reverse 1D Array(array=w4297) -> (reversed array=w4296:dbl[])
        }
        n2819 = for {
          tunnel: w4262 -> [w4305] mode=indexing
          tunnel: [w4304] -> w4261 mode=indexing
          workers-P: _ -> [_]
          n2820 = Reverse 1D Array(array=w4305) -> (reversed array=w4304:dbl[])
        }
        n2821 = for {
          tunnel: w4266 -> [w4307] mode=indexing
          tunnel: [w4306] -> w4265 mode=indexing
          workers-P: _ -> [_]
          n2822 = Reverse 1D Array(array=w4307) -> (reversed array=w4306:dbl[])
        }
        n2823 = for {
          tunnel: w4248 -> [w4301] mode=indexing
          tunnel: [w4300] -> w4247 mode=indexing
          workers-P: _ -> [_]
          n2824 = Reverse 1D Array(array=w4301) -> (reversed array=w4300:dbl[])
        }
        n2825 = for {
          tunnel: w4255 -> [w4303] mode=indexing
          tunnel: [w4302] -> w4254 mode=indexing
          workers-P: _ -> [_]
          n2826 = Reverse 1D Array(array=w4303) -> (reversed array=w4302:dbl[])
        }
        n2827 = Index Array(array=w4267, index (row)=0) -> (element=→"Waveform Graph":dbl[])  [unwired: 1 in]
        n2828 = Add(x=w4193, y=w4192) -> (x+y=w4179:dbl[][])
        n2829 = Add(x=w4166, y=w4165) -> (x+y=w4152:dbl[][])
        n2830 = Add(x=w4261, y=w4260) -> (x+y=w4259:dbl[][])
        n2831 = Add(x=w4265, y=w4264) -> (x+y=w4239:dbl[][])
        n2832 = Add(x=w4247, y=w4246) -> (x+y=w4245:dbl[][])
        n2833 = Add(x=w4254, y=w4253) -> (x+y=w4252:dbl[][])
        n2834 = Divide(x=w4245, y=2) -> (x/y=w4243:dbl[][])
        n2835 = Divide(x=w4259, y=2) -> (x/y=w4204:dbl[][])
        n2836 = To Single Precision Float(number=w4239) -> (single precision float=w4238:sgl[][])
        n2837 = To Single Precision Float(number=w4179) -> (single precision float=w4183:sgl[][])
        n2838 = To Single Precision Float(number=w4152) -> (single precision float=w4156:sgl[][])
        n2839 = Divide(x=w4252, y=2) -> (x/y=w4206:dbl[][])
        n2840 = Transpose 2D Array(2D array=w4243) -> (transposed array=→"Data map":dbl[][])
        n2841 = To Single Precision Float(number=w4204) -> (single precision float=w4210:sgl[][])
        n2842 = To Single Precision Float(number=w4206) -> (single precision float=w4207:sgl[][])
        n2843 = call "IMAQ ArrayToImage"("Image Pixels (Float)"=w4238, "Image"=w4176) -> ("Image Out"=w4241:T2)  [unwired: 8 in, 1 out]
        n2844 = call "IMAQ ArrayToImage"("Image Pixels (Float)"=w4183, "Image"=w4175) -> ("Image Out"=w4185:T2)  [unwired: 8 in, 1 out]
        n2845 = call "IMAQ ArrayToImage"("Image Pixels (Float)"=w4156, "Image"=w4148) -> ("Image Out"=w4158:T2)  [unwired: 8 in, 1 out]
        n2846 = call "IMAQ ArrayToImage"("Image Pixels (Float)"=w4210, "Image"=w4149) -> ("Image Out"=w4212:T2)  [unwired: 8 in, 1 out]
        n2847 = call "IMAQ Symmetry"("Type of Symmetry"=w4240, "Image Src"=w4241) -> ("Image Dst Out"=w4236:T2)  [unwired: 3 in, 1 out]
        n2848 = call "IMAQ ArrayToImage"("Image Pixels (Float)"=w4207, "Image"=w4150) -> ("Image Out"=w4209:T2)  [unwired: 8 in, 1 out]
        n2849 = call "IMAQ Symmetry"("Type of Symmetry"=w4184, "Image Src"=w4185) -> ("Image Dst Out"=w4181:T2)  [unwired: 3 in, 1 out]
        n2850 = call "IMAQ Symmetry"("Type of Symmetry"=w4157, "Image Src"=w4158) -> ("Image Dst Out"=w4154:T2)  [unwired: 3 in, 1 out]
        n2851 = call "IMAQ Symmetry"("Type of Symmetry"=w4211, "Image Src"=w4212) -> ("Image Dst Out"=→"Detection Laser X":T2)  [unwired: 3 in, 1 out]
        n2852 = call "IMAQ Symmetry"("Type of Symmetry"=w4208, "Image Src"=w4209) -> ("Image Dst Out"=→"Detection Laser Y":T2)  [unwired: 3 in, 1 out]
        n2853 = call "IMAQ Set Simple Calibration"("Calibration Axis Info"=T39 {"Origin Pixel"={"X"=0.0, "Y"=0.0}, "Angle Relative to Horizontal (deg)"=0.0, "Axis Reference"=0}, "Grid Descriptor"=T40 {"X Step"=0.3, "Y Step"=0.3, "Unit"=enum."Undefined"}, "Image"=w4236) -> ("Calibrated Image"=→"APD 1":T2)  [unwired: 7 in, 1 out]
        n2854 = call "IMAQ Set Simple Calibration"("Calibration Axis Info"=T39 {"Origin Pixel"={"X"=0.0, "Y"=0.0}, "Angle Relative to Horizontal (deg)"=0.0, "Axis Reference"=0}, "Grid Descriptor"=T40 {"X Step"=0.3, "Y Step"=0.3, "Unit"=enum."Undefined"}, "Image"=w4181) -> ("Calibrated Image"=→"APD 2":T2)  [unwired: 7 in, 1 out]
        n2855 = call "IMAQ Set Simple Calibration"("Calibration Axis Info"=T39 {"Origin Pixel"={"X"=0.0, "Y"=0.0}, "Angle Relative to Horizontal (deg)"=0.0, "Axis Reference"=0}, "Grid Descriptor"=T40 {"X Step"=0.3, "Y Step"=0.3, "Unit"=enum."Undefined"}, "Image"=w4154) -> ("Calibrated Image"=→"APD 3":T2)  [unwired: 7 in, 1 out]
      }
    }
    n2856 = case "For computing FFTs for display" shown="True" "Compute FFT" {
      tunnel: w3653 -> [_ w4779]
      frame False {
      }
      frame True {
        n2857 = Build Array("FFT 1 Choice 1", "FFT 1 Choice 2", "FFT 2 Choice 1", "FFT 2 Choice 2") -> (w4772:u16[])
        n2858 = Array Size(array=w4779) -> (size(s)=w4778:i32)
        n2859 = feedback-in #20(w4772) -> ()
        n2860 = feedback #20(u16[] [100, 100, 100, 100]) -> (w4773:u16[])
        n2861 = feedback-in #21("# Spectra to Ave.") -> ()
        n2862 = feedback #21("# Spectra to Ave.") -> (w4770:dbl)
        n2863 = Not Equal?(x="# Spectra to Ave.", y=w4770) -> (x != y?=w4769:bool)
        n2864 = Not Equal?(x=w4772, y=w4773) -> (x != y?=w4771:bool)
        n2865 = feedback #22(1.0) -> (w4756:dbl)
        n2866 = Compound Arithmetic op=OR("Reset FFT", w4771, w4769) -> (w4754:bool)
        n2867 = Select(t=1.0, s=w4754, f=w4756) -> (s? t:f=w4758:dbl)
        n2868 = Greater?(x=w4758, y="# Spectra to Ave.") -> (0:w4777:bool)
        n2869 = Increment(x=w4758) -> (x+1=w4757:dbl)
        n2870 = feedback-in #22(w4757) -> ()
        n2871 = local read "DMA Update Period (s)"() -> (w4752:dbl)
        n2872 = Multiply(x="# Spectra to Ave.", y=w4752) -> (x*y=→"Ave. Time (s)":dbl)
        n2873 = Build Array(cluster{"f0":dbl, "df":dbl, "magnitude":dbl[]} {"f0"=0.0, "df"=0.0, "magnitude"=[]} ("PSD")) -> (w4761:cluster{"f0":dbl, "df":dbl, "magnitude":dbl[]}[])
        n2874 = Build Array(w4761, w4761, w4761, w4761) -> (w4763:T49)
        n2875 = feedback #23(w4763) -> (w4768:T49)
        n2876 = for {
          N: 4 -> [_]
          tunnel: w4772 -> [w4801] mode=indexing
          tunnel: w4779 -> [w4802]
          tunnel: w4778 -> [w4804]
          tunnel: w4754 -> [w4797]
          tunnel: w4777 -> [w4796]
          tunnel: "# Spectra to Ave." -> [w4795]
          tunnel: [w4794] -> w4767 mode=indexing
          tunnel: w4768 -> [w4799] mode=indexing
          tunnel: [w4798] -> w4755 mode=indexing
          tunnel: w4758 -> [w4793]
          n2877 = Less?(x=w4801, y=w4804) -> (x < y?=w4803:bool)
          n2878 = Index Array(array=w4802, index=w4801) -> (element=w4800:waveform(dbl))
          n2879 = case shown="True" w4803 {
            tunnel: w4800 -> [_ w4821]
            tunnel: w4799 -> [w4806 w4819]
            tunnel: [w4806 w4807] -> w4798
            tunnel: w4797 -> [_ w4818]
            tunnel: w4796 -> [_ w4811]
            tunnel: w4795 -> [_ w4810]
            tunnel: [cluster{"f0":dbl, "df":dbl, "magnitude":dbl[]} {"f0"=0.0, "df"=0.0, "magnitude"=[]} ("PSD") w4812] -> w4794
            tunnel: w4793 -> [_ w4809]
            frame False {
            }
            frame True {
              n2880 = call <vilib>:"Std Deviation and Variance.vi"("X"=w4821) -> ("mean"=w4822:dbl)  [unwired: 1 in, 2 out]
              n2881 = Subtract(x=w4821, y=w4822) -> (x-y=w4820:waveform(dbl))
              n2882 = xnode "Spectral Measurements"("Signals"=w4820) -> ("PSD"=w4814:cluster{"f0":dbl, "df":dbl, "magnitude":dbl[]})  [unwired: 1 in, 1 out]
              n2883 = case shown="False" w4818 {
                tunnel: w4819 -> [w4831 _]
                tunnel: [w4827 w4836] -> w4807
                tunnel: w4814 -> [w4830 w4837]
                tunnel: w4811 -> [w4829 _]
                frame False {
                  n2884 = Build Array (concatenate)(w4831, w4830) -> (w4828:cluster{"f0":dbl, "df":dbl, "magnitude":dbl[]}[])
                  n2885 = case shown="True" w4829 {
                    tunnel: w4828 -> [w4832 w4835]
                    tunnel: [w4832 w4833] -> w4827
                    frame False {
                    }
                    frame True {
                      n2886 = Delete From Array(array=w4835, index=0) -> (array with subset deleted=w4833:cluster{"f0":dbl, "df":dbl, "magnitude":dbl[]}[])  [unwired: 1 in, 1 out]
                    }
                  }
                }
                frame True {
                  n2887 = Build Array(w4837) -> (w4836:cluster{"f0":dbl, "df":dbl, "magnitude":dbl[]}[])
                }
              }
              n2888 = for {
                tunnel: w4807 -> [w4826] mode=indexing
                tunnel: [w4825] -> w4817 mode=indexing
                workers-P: _ -> [_]
                n2889 = Unbundle By Name(w4826) -> ("magnitude"=w4825:dbl[])
              }
              n2890 = Transpose 2D Array(2D array=w4817) -> (transposed array=w4816:dbl[][])
              n2891 = for {
                tunnel: w4816 -> [w4824] mode=indexing
                tunnel: [w4823] -> w4815 mode=indexing
                workers-P: _ -> [_]
                n2892 = Add Array Elements(numeric array=w4824) -> (sum=w4823:dbl)
              }
              n2893 = Select(t=w4810, s=w4811, f=w4809) -> (s? t:f=w4808:dbl)
              n2894 = Divide(x=w4815, y=w4808) -> (x/y=w4813:dbl[])
              n2895 = Bundle By Name(cluster=w4814, "magnitude"=w4813) -> (w4812:cluster{"f0":dbl, "df":dbl, "magnitude":dbl[]})
            }
          }
        }
        n2896 = case shown="True" w4754 {
          tunnel: w4755 -> [w4786 w4792]
          tunnel: [w4786 w4787] -> w4753
          frame False {
          }
          frame True {
            n2897 = Array Subset(array=w4792, index (row)=0 ("index"), length (row)=4 ("length"), index (col)=0 ("index"), length (col)=1 ("length")) -> (w4787:T49)
          }
        }
        n2898 = feedback-in #23(w4753) -> ()
        n2899 = Split 1D Array(array=w4767, index=2) -> (first subarray=→"FFT 1":cluster{"f0":dbl, "df":dbl, "magnitude":dbl[]}[], second subarray=→"FFT 2":cluster{"f0":dbl, "df":dbl, "magnitude":dbl[]}[])
      }
    }
    n2900 = Index Array(array=w3651, index=4) -> (element=w3707:waveform(dbl))
    n2901 = Index Array(array=w3651, index=7) -> (element=w3704:waveform(dbl))
    n2902 = Divide(x="T1 offset_x (mV)", y=1000.0) -> (x/y=w3708:dbl)
    n2903 = feedback-in #24("Calibration") -> ()
    n2904 = feedback #24(u16 1 ("Calibration")) -> (w3726:u16)
    n2905 = Divide(x="T2 offset_x (mV)", y=1000.0) -> (x/y=w3706:dbl)
    n2906 = case shown="2" "Calibration" {
      tunnel: "T1 alpha_x (nm/V)" -> [_ w4100 w4121]
      tunnel: "T1 kappa_x (pN/nm)" -> [_ _ w4111]
      tunnel: "T2 alpha_x (nm/V)" -> [_ w4099 w4119]
      tunnel: "T2 kappa_x (pN/nm)" -> [_ _ w4112]
      tunnel: w3707 -> [w4082 w4097 w4117]
      tunnel: w3704 -> [w4081 w4095 w4115]
      tunnel: [w4082 w4094 w4114] -> w3735
      tunnel: [w4081 w4093 w4113] -> w3734
      tunnel: ["T1 X (V)" ("Label.Text") "T1 X (nm)" ("Label.Text") "T1 X (pN)" ("Label.Text")] -> w3723
      tunnel: ["T2 X (V)" ("Label.Text") "T2 X (nm)" ("Label.Text") "T2 X (pN)" ("Label.Text")] -> w3722
      tunnel: ["Position (V)" ("Label.Text") "Position (nm)" ("Label.Text") "Force (pN)" ("Label.Text")] -> w3724
      tunnel: w3706 -> [_ w4085 w4104]
      tunnel: w3708 -> [_ w4088 w4106]
      tunnel: ["Mean (V)" ("Label.Text") "Mean (nm)" ("Label.Text") "Mean (pN)" ("Label.Text")] -> w3719
      tunnel: ["Difference (V)" ("Label.Text") "Difference (nm)" ("Label.Text") "Difference (pN)" ("Label.Text")] -> w3659
      frame 0, Default {
      }
      frame 1 {
        n2907 = Unbundle By Name(w4097) -> ("Y"=w4101:dbl[])
        n2908 = Unbundle By Name(w4095) -> ("Y"=w4086:dbl[])
        n2909 = Subtract(x=w4101, y=w4088) -> (x-y=w4089:dbl[])
        n2910 = Subtract(x=w4086, y=w4085) -> (x-y=w4087:dbl[])
        n2911 = Multiply(x=w4087, y=w4099) -> (x*y=w4096:dbl[])
        n2912 = Multiply(x=w4100, y=w4089) -> (x*y=w4098:dbl[])
        n2913 = Bundle By Name(cluster=w4095, "Y"=w4096) -> (w4093:waveform(dbl))
        n2914 = Bundle By Name(cluster=w4097, "Y"=w4098) -> (w4094:waveform(dbl))
      }
      frame 2 {
        n2915 = Unbundle By Name(w4117) -> ("Y"=w4122:dbl[])
        n2916 = Unbundle By Name(w4115) -> ("Y"=w4120:dbl[])
        n2917 = Subtract(x=w4120, y=w4104) -> (x-y=w4105:dbl[])
        n2918 = Subtract(x=w4122, y=w4106) -> (x-y=w4107:dbl[])
        n2919 = Compound Arithmetic op=MULTIPLY(w4105, w4119, w4112) -> (w4116:dbl[])
        n2920 = Compound Arithmetic op=MULTIPLY(w4111, w4121, w4107) -> (w4118:dbl[])
        n2921 = Bundle By Name(cluster=w4115, "Y"=w4116) -> (w4113:waveform(dbl))
        n2922 = Bundle By Name(cluster=w4117, "Y"=w4118) -> (w4114:waveform(dbl))
      }
    }
    n2923 = case shown="True" "Read Lateness and Rel Phase" {
      tunnel: w3525 -> [w4037 w4070]
      tunnel: w3524 -> [w4038 w4069]
      tunnel: [w4037 w4042] -> w3701
      tunnel: [w4038 w4041] -> w3700
      frame False {
      }
      frame True {
        n2924 = xnode "Read/Write Control"("FPGA VI Reference In"=w4070, "error in"=w4069) -> ("FPGA VI Reference Out"=w4044:T20, "error out"=w4043:errorcluster, "GI Relative phase"=→"GI relative phase":i16, "Relative phase"=→"Relative phase (AI1)":i16, "AI Late Counter"=→"Late Counter (AI1)":u8, "GI Late Counter"=→"GI Late Counter":u8, "MCL Late Counter"=→"MCL Late Counter":u8, "MCL Relative Phase"=→"Relative Phase (MCL)":i16, "APD Acq Relative Phase"=→"APD Acq Relative Phase":i16, "APD 1 Gate Relative Phase"=→"APD 1 Gate Relative Phase":i16, "APD 2 Gate Relative Phase"=→"APD 2 Gate Relative Phase":i16, "APD Acq Late Counter"=→"APD Acq Late Counter":u8, "APD 1 Gate Late Counter"=→"APD 1 Gate Late Counter":u8, "APD 2 Gate Late Counter"=→"APD 2 Gate Late Counter":u8, "Green FB Relative Phase"=→"Relative phase (Green FB)":i16, "GI Relative phase 2"=→"GI relative phase 2":i16, "GI Late Counter 2"=→"GI Late Counter 2":u8, "Trap Pos FIFO Timeout"=→"Trap Pos FIFO Timeout":u16, "Trap AI FIFO Timeout"=→"Trap AI FIFO Timeout":u16, "RI Late Counter"=→"RI Late Counter":u8, "RI Relative phase"=→"RI relative phase":i16, "Green Late Counter"=→"Green AI Late Counter":u8, "BI Late Counter (AO)"=→"Late Counter (BI AO)":u8, "Blue Late Counter (D)"=→"Late Counter (BI DO)":u8, "BI Relative phase (AO)"=→"Relative phase (BI AO)":i16, "BI Relative phase (D)"=→"Relative phase (BI DO)":i16)